vi "Trajectory Builder.vi"() -> ()   [LabVIEW 2025] (continued)
        n148 = call "Versioned Write.vi"("Path Stuff"=w308, "Filename"="Filename", "Bordeaux paths in"=w327) -> ()  [unwired: 9 in]
        n149 = Bundle("Trajectory Data"=w329, "Updated Waypoints"=w330, w328, "sorted array out"=w316) -> (w339:T27)  [unwired: 1 in]
      }
      event "Open Command": Value Change {
        # "Open Panel button was pressed. Open the subVI for the selected command"
        n150 = event-data() -> ()  [unwired: 1 in, 1 out]
        n151 = Unbundle(w372) -> ("Updated Waypoints"=w371:cluster{"x":dbl, "y":dbl, "th":dbl}[])  [unwired: 3 out]
        n152 = Unbundle(w361) -> ("Filtered Command Info Out"=w360:T2)  [unwired: 2 out]
        n153 = call "Open Command Panel.vi"("Cached Commands"=w360, "Commands"=w370, "Tag"="Command Sequence") -> ("Found"=w367:bool)  [unwired: 8 in]
        n154 = Select(t="Command Sequence", s=w367, f="") -> (s? t:f=w364:string)
        n155 = Bundle(cluster=w368, "Filename"=w364) -> (w369:T18)  [unwired: 2 in]
      }
      event "Directory": Value Change {
        # "Negate timeout to immed update list of files"
        # "Directory button was pressed. Put up a file dialog to let the user choose a new directory for loading and saving paths.\nUpdate the titlebar."
        n156 = event-data() -> ()  [unwired: 1 in, 1 out]
        n157 = Unbundle(w387) -> ("Updated Waypoints"=w386:cluster{"x":dbl, "y":dbl, "th":dbl}[])  [unwired: 3 out]
        n158 = call "File Dialog"("start path"=w382, "prompt"="Path Folder", "button label"="Select") -> ("selected path"=w381:path, "error out"=w383:errorcluster)  [unwired: 9 in, 2 out]
        n159 = Select(t=w382, s=w383, f=w381) -> (s? t:f=w375:path)
        n160 = call "Change Paths Directory.vi"("VI Refnum"=w374, "config path"=w376, "Bordeaux paths directory"=w375) -> ()  [unwired: 8 in, 1 out]
      }
      event "Delete": Value Change {
        n161 = event-data() -> ()  [unwired: 1 in, 6 out]
        n162 = Unbundle(w397) -> ("Updated Waypoints"=w396:cluster{"x":dbl, "y":dbl, "th":dbl}[])  [unwired: 3 out]
        n163 = local read "Open"() -> (w392:i32[])
        n164 = property on="Open" class="MCListbox (strict)"() -> ("ItemNames"=w394:string[][])  [unwired: 2 in, 2 out]
        n165 = Array Size(array=w392) -> (size(s)=w391:i32)
        n166 = Index Array(array=w392) -> (element=w393:i32)  [unwired: 1 in]
        n167 = Array Subset(array=w394, index (row)=w393, length (row)=w391) -> (w390:string[][])  [unwired: 2 in]
        n168 = for {
          tunnel: w390 -> [w410] mode=indexing
          tunnel: w395 -> [w411]
          n169 = Index Array(array=w410, index=0) -> (element=w404:string)
          n170 = String To Path(string=w404) -> (path=w405:path)
          n171 = Build Path(base path=w411, name or relative path=w405) -> (appended path=w408:path)
          n172 = Delete(path (use dialog)=w408, confirm (F)=FALSE) -> (error out=w406:errorcluster)  [unwired: 3 in, 2 out]
          n173 = call <vilib>:"Clear Errors.vi"("error in (no error)"=w406) -> ()  [unwired: 5 in, 2 out]
        }
      }
      event "Open": Shortcut Menu Selection (User) {
        n174 = event-data() -> ("ItemTag"=w420:string)  [unwired: 1 in, 7 out]
        n175 = case shown="\"False\", Default" w420 {
          tunnel: w419 -> [_ _ w437 _]
          tunnel: w418 -> [w427 w430 w434 w450]
          tunnel: [w426 w429 w433 w449] -> w417
          tunnel: w415 -> [w425 w428 w432 _]
          tunnel: [w425 w428 w432 w449] -> w414
          frame "False", Default {
            n176 = Unbundle(w427) -> ("Updated Waypoints"=w426:cluster{"x":dbl, "y":dbl, "th":dbl}[])  [unwired: 3 out]
          }
          frame "New Path" {
            n177 = Unbundle(w430) -> ("Updated Waypoints"=w429:cluster{"x":dbl, "y":dbl, "th":dbl}[])  [unwired: 3 out]
            n178 = local write "Conditions"(T10 {"vInitial (fps)"=0.0, "vFinal (fps)"=0.0} ("Conditions")) -> ()
          }
          frame "Delete Path(s)" {
            n179 = local read "Open"() -> (w435:i32[])
            n180 = Unbundle(w434) -> ("Updated Waypoints"=w433:cluster{"x":dbl, "y":dbl, "th":dbl}[])  [unwired: 3 out]
            n181 = property on="Open" class="MCListbox (strict)"() -> ("ItemNames"=w436:string[][])  [unwired: 2 in, 2 out]
            n182 = Array Size(array=w435) -> (size(s)=w439:i32)
            n183 = Index Array(array=w435) -> (element=w440:i32)  [unwired: 1 in]
            n184 = Array Subset(array=w436, index (row)=w440, length (row)=w439) -> (w438:string[][])  [unwired: 2 in]
            n185 = for {
              tunnel: w438 -> [w447] mode=indexing
              tunnel: w437 -> [w448]
              n186 = Index Array(array=w447, index=0) -> (element=w441:string)
              n187 = String To Path(string=w441) -> (path=w442:path)
              n188 = Build Path(base path=w448, name or relative path=w442) -> (appended path=w445:path)
              n189 = Delete(path (use dialog)=w445, confirm (F)=FALSE) -> (error out=w443:errorcluster)  [unwired: 3 in, 2 out]
              n190 = call <vilib>:"Clear Errors.vi"("error in (no error)"=w443) -> ()  [unwired: 5 in, 2 out]
            }
          }
          frame "Append to Path" {
            n191 = local read "Limits"() -> (w459:T9)
            n192 = Unbundle(w450) -> ("Updated Waypoints"=w452:cluster{"x":dbl, "y":dbl, "th":dbl}[])  [unwired: 3 out]
            n193 = local read "Conditions"() -> (w460:T10)
            n194 = Unbundle(w459) -> ("Velocity (fps)"=w454:dbl, "Accel (fps^2)"=w453:dbl)  [unwired: 2 out]
            n195 = Delete From Array(array=w452) -> (deleted portion=w457:cluster{"x":dbl, "y":dbl, "th":dbl})  [unwired: 2 in, 1 out]
            n196 = Divide(x=w454, y=w453) -> (x/y=w458:dbl)
            n197 = Build Array(w457) -> (w456:cluster{"x":dbl, "y":dbl, "th":dbl}[])
            n198 = Unbundle(w460) -> ("vFinal (fps)"=w455:dbl)  [unwired: 1 out]
            n199 = call "Add First Point.vi"("Accel (f/s^2)"=w453, "Time (s)"=w458, "Initial Points"=w456) -> ("Points"=w449:cluster{"x":dbl, "y":dbl, "th":dbl}[])  [unwired: 8 in]
            n200 = Bundle("vFinal (fps)"=w455, 0.0) -> (w461:cluster{"vFinal (fps)":dbl, dbl})  [unwired: 1 in]
            n201 = local write "Conditions"(w461) -> ()
          }
        }
      }
      event "Open": Double Click {
        # "When a path file is double clicked, load it and update the controls/indicators on the panel"
        n202 = event-data() -> ("Row"=w466:i32)  [unwired: 1 in, 8 out]
        n203 = property on="Open" class="MCListbox (strict)"() -> ("ItemNames"=w491:string[][])  [unwired: 2 in, 2 out]
        n204 = Index Array(array=w491, index (row)=w466, index (col)=0) -> (element=w467:string)
        n205 = Build Path(base path=w472, name or relative path=w467) -> (appended path=w490:path)
        n206 = local write "Filename"(w467) -> ()
        n207 = call "Versioned Load.vi"("path"=w490) -> ("Trajectory Meta"=w471:cluster{"Drive Type":T11, "Path Type":T7}, "Current Limit"=w465:dbl, "Points out"=w473:cluster{"x":dbl, "y":dbl, "th":dbl}[], "Fields"=w478:T28, "Commands out"=w484:cluster{"Time (s)":dbl, T3, bool}[], "Zero V"=w479:bool, "Ball Pickup"=w464:bool, "Reversals"=w483:T25, "Trajectory Data"=w489:T12, "Zero Translational Velocity"=w463:bool, "Correct at Beginning \nof Path"=w462:bool)  [unwired: 15 in, 1 out]
        n208 = Unbundle(w483) -> ("Robot Backwards"=w482:bool, "Reverse Path"=w481:bool)
        n209 = Unbundle(w478) -> ("Sample Period (s)"=w477:dbl, w476:T29, "Conditions"=w475:T10, "Overrides"=w474:T8)  [unwired: 1 out]
        n210 = Unbundle(w471) -> ("Drive Type"=w470:T11, "Path Type"=w469:T7)
        n211 = local write "Correct at Beginning \nof Path"(w462) -> ()
        n212 = local write "Zero Translational\n Velocity"(w463) -> ()
        n213 = local write "Current Limit"(w465) -> ()
        n214 = local write "Robot Backwards"(w482) -> ()
        n215 = local write "Zero Velocity"(w479) -> ()
        n216 = local write "Reverse Path"(w481) -> ()
        n217 = local write "Pickup Balls"(w464) -> ()
        n218 = local write "Limits"(w476) -> ()
        n219 = local write "Drive Type"(w470) -> ()
        n220 = local write "Path Type"(w469) -> ()
        n221 = local write "Sample Period (s)"(w477) -> ()
        n222 = local write "Overrides"(w474) -> ()
        n223 = local write "Conditions"(w475) -> ()
        n224 = Bundle("Trajectory Data"=w489, "Points out"=w473, "Fields"=w478, "Commands out"=w484) -> (w480:T30)  [unwired: 1 in]
      }
      event "Picture": Mouse Down {
        # "Object being clicked"
        # "Process a mouse down on the picture control. Only left clicks do anything.\nDetermine if any object was clicked on and mark it as the drag object for \nmouse move messages."
        n225 = event-data() -> ("Coords"=w506:T31, "Button"=w508:u16, "Mods"=w507:cluster{"Double Click":bool, "Menu Key":bool}, "PlatMods"=w503:T32)  [unwired: 1 in]
        n226 = Unbundle(w496) -> ("Drag Object"=w495:cluster{"Index":i32, "x":dbl, "y":dbl})  [unwired: 2 out]
        n227 = Unbundle(w500) -> ("Updated Waypoints"=w499:cluster{"x":dbl, "y":dbl, "th":dbl}[])  [unwired: 3 out]
        n228 = case shown="1" w508 {
          tunnel: w507 -> [_ _ w520]
          tunnel: w506 -> [_ _ w525]
          tunnel: w499 -> [w512 w516 w526]
          tunnel: [w512 w516 w530] -> w505
          tunnel: w504 -> [_ _ w527]
          tunnel: w495 -> [w510 w513 w521]
          tunnel: [w509 w515 w522] -> w497
          tunnel: w503 -> [_ _ w518]
          frame 0, Default {
            # "middle mouse?"
            n229 = Bundle(cluster=w510, "Index"=-1) -> (w509:cluster{"Index":i32, "x":dbl, "y":dbl})  [unwired: 2 in]
          }
          frame 2 {
            # "Right Button"
            n230 = Bundle(cluster=w513, "Index"=-1) -> (w515:cluster{"Index":i32, "x":dbl, "y":dbl})  [unwired: 2 in]
          }
          frame 1 {
            # "Left Button"
            n231 = Unbundle By Name(w520) -> ("Double Click"=w519:bool)
            n232 = property on="Picture" class="Pict"() -> ("Position"=w529:T16, "Draw Area Size"=w528:T33)  [unwired: 2 in, 2 out]
            n233 = Unbundle By Name(w518) -> ("Shift"=w517:bool)
            n234 = call "Point Test Shapes.vi"("Coords"=w525, "Points"=w526, "Picture in"=w527) -> ("Pt Test Results"=w524:enum16{"Miss", "Rect Hit", "Arrow Hit"}, "Results"=w523:T17)  [unwired: 7 in]
            n235 = case shown="\"Rect Hit\"" w524 {
              tunnel: w519 -> [_ _ w577]
              tunnel: w526 -> [w534 w562 w571]
              tunnel: w523 -> [_ w560 w578]
              tunnel: [w537 w563 w572] -> w530
              tunnel: w525 -> [w538 _ _]
              tunnel: w529 -> [w536 _ _]
              tunnel: w528 -> [w535 _ _]
              tunnel: [w532 w555 w574] -> w522
              tunnel: w521 -> [w531 _ w575]
              tunnel: w517 -> [w533 _ w567]
              frame "Miss", Default {
                n236 = case shown="True" w533 {
                  tunnel: w538 -> [w550 _]
                  tunnel: [w547 w554] -> w537
                  tunnel: w536 -> [w546 _]
                  tunnel: w535 -> [w545 _]
                  tunnel: w534 -> [w541 w554]
                  tunnel: [w540 w553] -> w532
                  tunnel: w531 -> [_ w551]
                  frame False {
                    n237 = call "Map to Feet.vi"("Draw Area Size"=w545, "Position"=w546, "Coords (px)"=w550) -> ("Point (ft)"=w544:cluster{dbl, dbl})  [unwired: 8 in]
                    n238 = Array Size(array=w541) -> (size(s)=w539:i32)
                    n239 = Unbundle(w544) -> (w543:dbl, w542:dbl)
                    n240 = Bundle(w543, w542, nan) -> (w548:cluster{dbl, dbl, dbl})  [unwired: 1 in]
                    n241 = Bundle(w539, w543, w542) -> (w540:cluster{i32, dbl, dbl})  [unwired: 1 in]
                    n242 = Build Array (concatenate)(w541, w548) -> (w547:cluster{"x":dbl, "y":dbl, "th":dbl}[])
                  }
                  frame True {
                    n243 = Bundle(cluster=w551, "Index"=-1) -> (w553:cluster{"Index":i32, "x":dbl, "y":dbl})  [unwired: 2 in]
                  }
                }
              }
              frame "Arrow Hit" {
                # "start tracking rotation"
                n244 = Unbundle(w560) -> ("Index"=w559:i32)  [unwired: 1 out]
                n245 = Index Array(array=w562, index=w559) -> (element=w561:cluster{"x":dbl, "y":dbl, "th":dbl})
                n246 = Unbundle(w561) -> ("x"=w558:dbl, "y"=w557:dbl, "th"=w565:dbl)
                n247 = Bundle(cluster=w561, "th"=w565) -> (w564:cluster{"x":dbl, "y":dbl, "th":dbl})  [unwired: 2 in]
                n248 = Bundle(-2, "x"=w558, "y"=w557) -> (w555:cluster{i32, "x":dbl, "y":dbl})  [unwired: 1 in]
                n249 = Replace Array Subset(array=w562, new element=w564) -> (w563:cluster{"x":dbl, "y":dbl, "th":dbl}[])  [unwired: 1 in]
              }
              frame "Rect Hit" {
                n250 = Unbundle(w578) -> ("Index"=w576:i32)  [unwired: 1 out]
                n251 = Array Size(array=w571) -> (size(s)=w570:i32)
                n252 = Greater?(x=w570, y=2) -> (0:w568:bool)
                n253 = And(x=w567, y=w568) -> (x .and. y?=w566:bool)
                n254 = case shown="True" w566 {
                  tunnel: w577 -> [w582 _]
                  tunnel: w576 -> [w581 w585]
                  tunnel: [w580 -1 ("length")] -> w573
                  tunnel: w571 -> [w579 w588]
                  tunnel: [w579 w587] -> w572
                  frame False {
                    n255 = case shown="False" w582 {
                      tunnel: w581 -> [w583 _]
                      tunnel: [w583 -1] -> w580
                      frame False {
                      }
                      frame True {
                        # "TODO Toggle last pt"
                      }
                    }
                  }
                  frame True {
                    n256 = case shown="0" w585 {
                      tunnel: w588 -> [w589 w593]
                      tunnel: w585 -> [_ w592]
                      tunnel: [w589 w590] -> w587
                      frame 0 {
                      }
                      frame Default {
                        n257 = Delete From Array(array=w593, length=1, index=w592) -> (array with subset deleted=w590:cluster{"x":dbl, "y":dbl, "th":dbl}[])  [unwired: 1 out]
                      }
                    }
                  }
                }
                n258 = Bundle(cluster=w575, "Index"=w573) -> (w574:cluster{"Index":i32, "x":dbl, "y":dbl})  [unwired: 2 in]
              }
            }
          }
        }
        n259 = Bundle(cluster=w496, "Drag Object"=w497) -> (w498:T18)  [unwired: 2 in]
      }
      event "Picture": Mouse Move; "Picture": Mouse Up {
        # "If an object was clicked on and is being moved, update position.\nIf nothing is being dragged, you may be hovering over an object and\nwant to draw it differently."
        n260 = event-data() -> ("Type"=w619:T21, "Coords"=w621:T31)  [unwired: 1 in]
        n261 = local read "Robot Size (in)"() -> (w601:cluster{"width":dbl, "height":dbl})
        n262 = Index Array(array=w595) -> (element=w596:cluster{"width":dbl, "height":dbl})  [unwired: 1 in]
        n263 = Unbundle By Name(w601) -> ("width"=w599:dbl)
        n264 = Unbundle By Name(w596) -> ("width"=w594:dbl)  [unwired: 1 out]
        n265 = Divide(x=w599, y=24.0) -> (x/y=w598:dbl)
        n266 = Subtract(x=w594, y=w598) -> (x-y=w597:dbl)
        n267 = Unbundle(w615) -> ("Updated Waypoints"=w614:cluster{"x":dbl, "y":dbl, "th":dbl}[])  [unwired: 3 out]
        n268 = Unbundle(w607) -> ("Drag Object"=w610:cluster{"Index":i32, "x":dbl, "y":dbl})  [unwired: 2 out]
        n269 = Unbundle(w610) -> ("Index"=w618:i32)  [unwired: 2 out]
        n270 = case shown="Default" w618 {
          selector: w618 -> [w632 _]
          tunnel: w621 -> [w641 w649]
          tunnel: [w639 w648] -> w612
          tunnel: [w636 w647] -> w620
          tunnel: w614 -> [w637 w647]
          tunnel: [w633 w646] -> w613
          tunnel: w610 -> [w624 w646]
          tunnel: w619 -> [w634 _]
          tunnel: "Snap to foot" -> [w629 _]
          tunnel: "Snap robot to baseline" -> [w630 _]
          tunnel: "Angle Limiter" -> [w631 _]
          tunnel: w606 -> [w623 w645]
          tunnel: w605 -> [_ w644]
          tunnel: w597 -> [w622 _]
          frame Default {
            # "Mouse up changes indes to break tracking,\notherwise update coords"
            n271 = property on="Picture" class="Pict"() -> ("Position"=w642:T16, "Draw Area Size"=w643:T33)  [unwired: 2 in, 2 out]
            n272 = Bundle("Snap robot to baseline"=w630, "Snap to foot"=w629, "Angle Limiter"=w631) -> (w628:T34)  [unwired: 1 in]
            n273 = Equal?(x=lveventtype."Mouse Up" ("Type"), y=w634) -> (x = y?=w627:bool)
            n274 = call "Map to Feet.vi"("Draw Area Size"=w643, "Position"=w642, "Coords (px)"=w641) -> ("Point (ft)"=w640:cluster{dbl, dbl})  [unwired: 8 in]
            n275 = call "Handle Pos and Rot.vi"("Starting Line Y"=w622, "Mouse Up"=w627, "Picture in"=w623, "Option"=w628, "Coord (ft)"=w640, "Index"=w632, "Points in"=w637) -> ("Points out"=w636:cluster{"x":dbl, "y":dbl, "th":dbl}[])  [unwired: 4 in]
            n276 = Bundle(cluster=w624, "Index"=-1) -> (w625:cluster{"Index":i32, "x":dbl, "y":dbl})  [unwired: 2 in]
            n277 = Bundle(w632, "Pt Test Results"=enum16{"Miss", "Rect Hit", "Arrow Hit"}."Rect Hit") -> (w639:T35)  [unwired: 1 in]
            n278 = Select(t=w625, s=w627, f=w624) -> (s? t:f=w633:cluster{"Index":i32, "x":dbl, "y":dbl})
          }
          frame -1 {
            n279 = call "Point Test Shapes.vi"("Array"=w644, "Coords"=w649, "Points"=w647, "Picture in"=w645) -> ("Results"=w648:T17)  [unwired: 6 in, 1 out]
          }
        }
        n280 = Bundle(cluster=w607, "Drag Object"=w613, "Hover Object"=w612) -> (w611:T18)  [unwired: 1 in]
      }
      event "Origin Reflection", "Sample Period (s)", "Horizontal Reflection", "Conditions", "Vertical Reflection": Value Change {
        # "Don't updates pts to fit rules"
        # "Changes to any of these controls will update the picture and other indicators to be consistent."
        n281 = event-data() -> ("CtlRef"=w657:refnum<vi>)  [unwired: 1 in]
        n282 = control-ref of="Vertical Reflection"() -> (w665:refnum<vi>)
        n283 = control-ref of="Origin Reflection"() -> (w658:refnum<vi>)
        n284 = control-ref of="Horizontal Reflection"() -> (w678:refnum<vi>)
        n285 = Index Array(array=w661) -> (element=w660:cluster{"width":dbl, "height":dbl})  [unwired: 1 in]
        n286 = Unbundle By Name(w660) -> ("width"=w659:dbl, "height"=w655:dbl)
        n287 = Equal?(x=w657, y=w658) -> (x = y?=w656:bool)
        n288 = Equal?(x=w678, y=w657) -> (x = y?=w663:bool)
        n289 = Equal?(x=w657, y=w665) -> (x = y?=w653:bool)
        n290 = Unbundle(w674) -> ("Updated Waypoints"=w654:cluster{"x":dbl, "y":dbl, "th":dbl}[])  [unwired: 3 out]
        n291 = case shown="True" w656 {
          tunnel: w654 -> [w679 w682]
          tunnel: [w679 w680] -> w651
          frame False {
          }
          frame True {
            n292 = Index Array(array=w682) -> (element=w681:cluster{"x":dbl, "y":dbl, "th":dbl})  [unwired: 1 in]
            n293 = for {
              tunnel: w682 -> [w700] mode=indexing
              tunnel: w681 -> [w699]
              tunnel: [w683] -> w680 mode=indexing
              n294 = Unbundle(w699) -> ("x"=w697:dbl, "y"=w695:dbl)  [unwired: 1 out]
              n295 = Unbundle(w700) -> ("x"=w693:dbl, "y"=w691:dbl, "th"=w690:dbl)
              n296 = Multiply(x=2.0, y=w697) -> (x*y=w694:dbl)
              n297 = Subtract(x=w694, y=w693) -> (x-y=w686:dbl)
              n298 = Add(x=w690, y=180.0) -> (x+y=w688:dbl)
              n299 = Multiply(x=2.0, y=w695) -> (x*y=w692:dbl)
              n300 = Quotient & Remainder(x=w688, y=360.0) -> (x-y*floor(x/y)=w684:dbl)  [unwired: 1 out]
              n301 = Subtract(x=w692, y=w691) -> (x-y=w685:dbl)
              n302 = Bundle(w686, w685, w684) -> (w683:cluster{dbl, dbl, dbl})  [unwired: 1 in]
            }
          }
        }
        n303 = case shown="True" w663 {
          tunnel: w654 -> [w716 w719]
          tunnel: [w716 w718] -> w664
          tunnel: w659 -> [_ w717]
          frame False {
          }
          frame True {
            n304 = for {
              tunnel: w719 -> [w729] mode=indexing
              tunnel: [w726] -> w718 mode=indexing
              tunnel: w717 -> [w723]
              n305 = Unbundle(w729) -> ("x"=w728:dbl, "y"=w727:dbl, "th"=w721:dbl)
              n306 = Negate(x=w728) -> (-x=w725:dbl)
              n307 = Subtract(x=180.0, y=w721) -> (x-y=w720:dbl)
              n308 = Add(x=w723, y=w725) -> (x+y=w724:dbl)
              n309 = Bundle(w724, "y"=w727, w720) -> (w726:cluster{dbl, "y":dbl, dbl})  [unwired: 1 in]
            }
          }
        }
        n310 = case shown="True" w653 {
          tunnel: w654 -> [w701 w704]
          tunnel: [w701 w703] -> w652
          tunnel: w655 -> [_ w702]
          frame False {
          }
          frame True {
            n311 = for {
              tunnel: w704 -> [w714] mode=indexing
              tunnel: [w715] -> w703 mode=indexing
              tunnel: w702 -> [w705]
              n312 = Unbundle By Name(w714) -> ("y"=w713:dbl, "x"=w712:dbl, "th"=w709:dbl)
              n313 = Negate(x=w713) -> (-x=w707:dbl)
              n314 = Negate(x=w709) -> (-x=w708:dbl)
              n315 = Add(x=w705, y=w707) -> (x+y=w706:dbl)
              n316 = Swap Values(12:w706, 14:w712) -> (1:w711:dbl, 3:w710:dbl)  [unwired: 1 in]
              n317 = Bundle(w711, w710, w708) -> (w715:cluster{dbl, dbl, dbl})  [unwired: 1 in]
            }
          }
        }
        n318 = Select(t=w652, s=w653, f=w651) -> (s? t:f=w650:cluster{"x":dbl, "y":dbl, "th":dbl}[])
        n319 = Select(t=w664, s=w663, f=w650) -> (s? t:f=w662:cluster{"x":dbl, "y":dbl, "th":dbl}[])
        n320 = local read "Path Type"() -> (w669:T7)
        n321 = case shown="\"Clothoid\", Default" w669 {
          tunnel: "Unjank" -> [_ w733]
          tunnel: w674 -> [_ w732]
          tunnel: "Turn Acceleration" -> [_ w731]
          tunnel: "Turn Deceleration" -> [_ w730]
          frame "Bezier" {
          }
          frame "Clothoid", Default {
            n322 = case shown="True" w733 {
              tunnel: w732 -> [_ w734]
              tunnel: w731 -> [_ w737]
              tunnel: w730 -> [_ w736]
              frame False {
              }
              frame True {
                n323 = call "Turn Smother.vi"("Ignore Deceleration"=w736, "Ignore Acceleration"=w737, "Internal Path Stuff"=w734) -> ("Overrides"=w735:T8)  [unwired: 1 in]
                n324 = local write "Overrides"(w735) -> ()
              }
            }
          }
        }
      }
      event Key Down?; event type 5.0.x8000000b {
        # "If hovering over an object, nudge using arrow keys"
        n325 = event-data() -> ("VKey"=w759:T36)  [unwired: 1 in]
        n326 = Index Array(array=w739) -> (element=w740:cluster{"width":dbl, "height":dbl})  [unwired: 1 in]
        n327 = local read "Robot Size (in)"() -> (w742:cluster{"width":dbl, "height":dbl})
        n328 = Unbundle By Name(w740) -> ("width"=w738:dbl)  [unwired: 1 out]
        n329 = Unbundle By Name(w742) -> ("width"=w744:dbl)
        n330 = Divide(x=w744, y=24.0) -> (x/y=w743:dbl)
        n331 = local read "Snap robot to baseline"() -> (w766:bool)
        n332 = Unbundle(w753) -> ("Updated Waypoints"=w752:cluster{"x":dbl, "y":dbl, "th":dbl}[])  [unwired: 3 out]
        n333 = Subtract(x=w738, y=w743) -> (x-y=w741:dbl)
        n334 = local read "Angle Limiter"() -> (w764:enum16{"90", "45", "15", "1"})
        n335 = local read "Snap to foot"() -> (w765:bool)
        n336 = Unbundle(w750) -> ("Hover Object"=w751:T17)  [unwired: 2 out]
        n337 = case shown="\"Up\"" w759 {
          tunnel: [cluster{dbl, dbl} {0.0, 0.0} ("Coord (ft)") cluster{dbl, dbl} {0.0, 0.1} ("Coord (ft)") cluster{dbl, dbl} {0.0, -0.1} ("Coord (ft)") cluster{dbl, dbl} {-0.1, 0.0} ("Coord (ft)") cluster{dbl, dbl} {0.1, 0.0} ("Coord (ft)")] -> w761
          tunnel: [_ w780 w782 w784 w786] -> w757
          tunnel: TRUE ("Delta") -> [_ w780 w782 w784 w786]
          frame Default {
          }
          frame "Up" {
          }
          frame "Down" {
          }
          frame "Left" {
          }
          frame "Right" {
          }
        }
        n338 = Unbundle(w751) -> ("Index"=w749:i32, "Pt Test Results"=w758:enum16{"Miss", "Rect Hit", "Arrow Hit"})
        n339 = Bundle("Snap robot to baseline"=w766, "Snap to foot"=w765, "Angle Limiter"=w764) -> (w763:T34)  [unwired: 1 in]
        n340 = case shown="\"Rect Hit\", Default" w758 {
          tunnel: [w769 w778] -> w767
          tunnel: w754 -> [_ w777]
          tunnel: w763 -> [_ w776]
          tunnel: w752 -> [w769 w775]
          tunnel: TRUE ("Delta") -> [_ w774]
          tunnel: w761 -> [_ w773]
          tunnel: w757 -> [_ w772]
          tunnel: [_ w772] -> w756
          tunnel: w749 -> [_ w771]
          tunnel: w741 -> [_ w770]
          frame "Miss" {
          }
          frame "Rect Hit", Default {
            n341 = call "Handle Pos and Rot.vi"("Starting Line Y"=w770, "Delta"=w774, "Picture in"=w777, "Option"=w776, "Coord (ft)"=w773, "Index"=w771, "Points in"=w775) -> ("Points out"=w778:cluster{"x":dbl, "y":dbl, "th":dbl}[])  [unwired: 4 in]
          }
        }
        n342 = event-data("Discard?"=w756) -> ()  [unwired: 1 in, 1 out]
      }
      event User Event {
        # "Fire events to animate the timeline\nuntil we reach the end"
        n343 = event-data() -> ("Data"=w802:i32)  [unwired: 1 in]
        n344 = Unbundle(w795) -> ("Updated Waypoints"=w794:cluster{"x":dbl, "y":dbl, "th":dbl}[])  [unwired: 3 out]
        n345 = Tick Count (ms)() -> (millisecond timer value=w805:u32)
        n346 = Subtract(x=w805, y=w802) -> (x-y=w804:u32)
        n347 = Multiply(x=w804, y=0.001) -> (x*y=w801:dbl)
        n348 = local read "Duration (s)"() -> (w788:dbl)
        n349 = Quotient & Remainder(x=w801, y=0.02) -> (floor(x/y)=w799:dbl)  [unwired: 1 out]
        n350 = Wait (ms)(milliseconds to wait=u32 50) -> ()  [unwired: 1 out]
        n351 = Multiply(x=0.02, y=w799) -> (x*y=w798:dbl)
        n352 = Less Or Equal?(x=w798, y=w788) -> (x <= y?=w807:bool)
        n353 = case shown="True" w807 {
          tunnel: w789 -> [_ w812]
          tunnel: w802 -> [_ w810]
          tunnel: w798 -> [_ w811]
          tunnel: w788 -> [w809 _]
          frame False {
            n354 = local write "Time (s)"(w809) -> ()
          }
          frame True {
            n355 = Generate User Event(user event=w812, event data cluster=w810) -> ()  [unwired: 2 in, 2 out]
            n356 = local write "Time (s)"(w811) -> ()
          }
        }
      }
      event "New Page Selector": Value Change {
        # "If looking at the commands, look at projects for one with a RIO target"
        n357 = event-data() -> ("NewVal"=w818:T1)  [unwired: 1 in]
        n358 = Unbundle(w821) -> ("Updated Waypoints"=w820:cluster{"x":dbl, "y":dbl, "th":dbl}[])  [unwired: 3 out]
        n359 = case shown="\"Command Sequencer\"" w818 {
          tunnel: [w824 w825] -> w814
          tunnel: w817 -> [w824 _]
          frame "Trajectory Settings", Default {
          }
          frame "Command Sequencer" {
            n360 = call "Find RT Projects.vi"() -> ("Paths"=w826:path[], "Targets"=w827:refnum<vi>[], "Project Names"=w828:string[])  [unwired: 9 in]
            n361 = property on="Projects" class="Ring (strict)"("Strings []"=w828) -> ()  [unwired: 2 in, 2 out]
            n362 = Bundle("Targets"=w827, "Paths"=w826) -> (w825:cluster{"Targets":refnum<vi>[], "Paths":path[]})  [unwired: 1 in]
          }
        }
        n363 = local write "Tab Control"("New Page Selector") -> ()
      }
      event "Refresh": Value Change {
        # "Refresh button was pressed. Reload the command info from the project.\nLater, maybe store this in a file because it takes awhile to recompute."
        n364 = event-data() -> ()  [unwired: 1 in, 1 out]
        n365 = Unbundle(w837) -> ("Updated Waypoints"=w836:cluster{"x":dbl, "y":dbl, "th":dbl}[])  [unwired: 3 out]
        n366 = flat-sequence {
          tunnel: [w840] -> w830
          tunnel: w832 -> [w847]
          tunnel: [w851] -> w831
          tunnel: w830 -> [w841]
          tunnel: [w841] -> w829
          tunnel: [w857] -> w834
          tunnel: w831 -> [w857]
          tunnel: w829 -> [w856]
          frame #0 {
            n367 = call <vilib>:"Set Busy.vi"() -> ("error out"=w840:errorcluster)  [unwired: 10 in, 1 out]
          }
          frame #1 {
            n368 = Unbundle(w847) -> ("Targets"=w846:refnum<vi>[], "Paths"=w845:path[])
            n369 = Index Array(array=w846, index="Projects") -> (element=w855:refnum<vi>)
            n370 = Index Array(array=w845, index="Projects") -> (element=w843:path)
            n371 = Strip Path(path=w843) -> (stripped path=w842:path)  [unwired: 1 out]
            n372 = global read "Global Settings.vi" "Icon Scale Factor"() -> (w848:dbl)
            n373 = call "Find Command Names.vi"("project root path"=w842, "TargetItem in"=w855) -> ("Paths"=w854:path[], "Command Info"=w853:T37)  [unwired: 8 in]
            n374 = call "Format Commands to Tree.vi"("Paths"=w854, "Command Info"=w853) -> ("2D Picture"=w852:picture, "Filtered Command Info Out"=w850:T2)  [unwired: 8 in]
            n375 = call "Resize Icons.vi"("Scale Factor"=w848, "Filtered Command Info Out"=w850) -> ("Filtered Command Info Out"=w849:T2)  [unwired: 9 in]
            n376 = Bundle("Filtered Command Info Out"=w849, "2D Picture"=w852, "stripped path"=w842) -> (w851:T38)  [unwired: 1 in]
            n377 = local write "Command Palette"(w852) -> ()
            n378 = local write "Cache"(w851) -> ()
          }
          frame #2 {
            n379 = call <vilib>:"Unset Busy.vi"("error in (no error)"=w856) -> ()  [unwired: 10 in, 1 out]
          }
        }
        n380 = call-poly <vilib>:"Set Cursor.vi"() -> ()  [unwired: 10 in, 2 out]
      }
      event "WayPoints": Value Change {
        # "If the waypoints control is hand-edited, pass the new data along to update the picture and other indicators\nand make it consistent"
        n381 = event-data() -> ("NewVal"=w858:cluster{"x":dbl, "y":dbl, "th":dbl}[])  [unwired: 1 in]
      }
      event event #0x53 {
        # "This is an alternative to the Inhale button. Notice that it doesn't actually modify anything at the\nmoment."
        n382 = event-data() -> ("VIName"=w868:string)  [unwired: 1 in]
        n383 = Unbundle(w878) -> ("Updated Waypoints"=w877:cluster{"x":dbl, "y":dbl, "th":dbl}[])  [unwired: 3 out]
        n384 = Unbundle(w876) -> ("Filename"=w867:string)  [unwired: 2 out]
        n385 = Search and Replace String(input string=w867, search string=w868, replace string=w868) -> (number of replacements=w873:i32)  [unwired: 5 in, 3 out]
        n386 = call "Find Command with Tag.vi"("Command Tag"=w867, "Commands"=w866) -> ("Index"=w874:i32, "Found Command"=w875:cluster{"Time (s)":dbl, T3, bool}, "Found"=w871:bool)  [unwired: 7 in]
        n387 = Not Equal To 0?(x=w873) -> (x != 0?=w872:bool)
        n388 = And(x=w871, y=w872) -> (x .and. y?=w870:bool)
        n389 = disable-structure shown="Disabled" {
          disable-tunnel: w875 -> [w886 _]
          disable-tunnel: w874 -> [w885 _]
          disable-tunnel: w870 -> [w884 _]
          disable-tunnel: [w883 _] -> w869
          disable-tunnel: w866 -> [w882 _]
          frame Disabled {
            n390 = case shown="True" w884 {
              tunnel: w886 -> [_ w893]
              tunnel: w885 -> [_ w900]
              tunnel: w882 -> [w887 w902]
              tunnel: [w887 w901] -> _
              tunnel: [_ FALSE] -> w883
              frame False {
              }
              frame True {
                n391 = Unbundle(w893) -> (w895:T3)  [unwired: 2 out]
                n392 = Unbundle(w895) -> ("Path"=w899:path)  [unwired: 6 out]
                n393 = Open VI Reference(vi path=w899) -> (vi reference=w897:refnum<vi>)  [unwired: 5 in, 1 out]
                n394 = property class="VI"(reference=w897) -> (reference out=w890:refnum<vi>, "Panel"=w898:refnum<vi>)  [unwired: 1 in, 1 out]
                n395 = property class="Pnl"(reference=w898) -> ("Controls[]"=w896:refnum<vi>[])  [unwired: 1 in, 2 out]
                n396 = for {
                  tunnel: w896 -> [w907] mode=indexing
                  tunnel: [w904] -> w894 mode=indexing
                  shift-right: [w903] -> w889
                  shift-left: w890 -> [w903]
                  n397 = property class="Ctl"(reference=w907) -> ("Label.Text"=w906:string, "Value"=w905:variant)  [unwired: 1 in, 2 out]
                  n398 = Bundle("Label.Text"=w906, "Value"=w905) -> (w904:cluster{"Label.Text":string, "Value":variant})  [unwired: 1 in]
                }
                n399 = Bundle(cluster=w895, "All Control Values Variant"=w894) -> (w892:T3)  [unwired: 6 in]
                n400 = Bundle(cluster=w893, w892) -> (w891:cluster{"Time (s)":dbl, T3, bool})  [unwired: 2 in]
                n401 = Replace Array Subset(array=w902, new element=w891, index=w900) -> (w901:cluster{"Time (s)":dbl, T3, bool}[])
                n402 = Close Reference(reference=w889) -> ()  [unwired: 1 in, 1 out]
              }
            }
          }
          frame Enabled {
          }
        }
      }
      event "Inhale": Value Change {
        # "Inhale button was pressed. Get the value of the controls/parameters and make them the\nvalues that will be used for the command."
        n403 = event-data() -> ()  [unwired: 1 in, 1 out]
        n404 = Unbundle(w919) -> ("Updated Waypoints"=w918:cluster{"x":dbl, "y":dbl, "th":dbl}[])  [unwired: 3 out]
        n405 = Unbundle(w917) -> ("Filename"=w916:string)  [unwired: 2 out]
        n406 = Unbundle(w910) -> ("Filtered Command Info Out"=w909:T2)  [unwired: 2 out]
        n407 = call "Find Command with Tag.vi"("Command Tag"=w916, "Commands"=w908) -> ("Index"=w913:i32, "Found Command"=w914:cluster{"Time (s)":dbl, T3, bool}, "Found"=w915:bool)  [unwired: 7 in]
        n408 = case shown="True" w915 {
          tunnel: w914 -> [_ w940]
          tunnel: w913 -> [_ w946]
          tunnel: w908 -> [w923 w948]
          tunnel: [w923 w947] -> w912
          tunnel: [_ TRUE] -> w911
          tunnel: w909 -> [_ w925]
          frame False {
          }
          frame True {
            n409 = Unbundle(w940) -> (w942:T3)  [unwired: 2 out]
            n410 = Unbundle(w942) -> ("Name"=w926:string, "Path"=w945:path)  [unwired: 5 out]
            n411 = Open VI Reference(vi path=w945) -> (vi reference=w927:refnum<vi>, error out=w931:errorcluster)  [unwired: 5 in]
            n412 = Unbundle(w931) -> ("code"=w930:i32)  [unwired: 2 out]
            n413 = Not Equal?(x=w930, y=0) -> (x != y?=w928:bool)
            n414 = case shown="False" w928 {
              tunnel: w927 -> [w949 w953]
              tunnel: w926 -> [_ w952]
              tunnel: w925 -> [_ w951]
              tunnel: [w949 w950] -> w924
              frame False {
              }
              frame True {
                n415 = call "Replace Command with Cached Command.vi"("Cached Commands"=w951, "Name"=w952, "VI in"=w953) -> ("VI out"=w950:refnum<vi>)  [unwired: 8 in]
              }
            }
            n416 = property class="VI"(reference=w924) -> (reference out=w937:refnum<vi>, "Panel"=w944:refnum<vi>)  [unwired: 1 in, 1 out]
            n417 = property class="Pnl"(reference=w944) -> (reference out=w935:refnum<vi>, "Controls[]"=w943:refnum<vi>[])  [unwired: 1 in, 1 out]
            n418 = for {
              tunnel: w943 -> [w959] mode=indexing
              tunnel: [w956] -> w941 mode=indexing
              shift-right: [w955] -> w934
              shift-left: w937 -> [w955]
              shift-right: [w954] -> _
              shift-left: w935 -> [w954]
              n419 = property class="Ctl"(reference=w959) -> ("Label.Text"=w958:string, "Value"=w957:variant)  [unwired: 1 in, 2 out]
              n420 = Bundle("Label.Text"=w958, "Value"=w957) -> (w956:cluster{"Label.Text":string, "Value":variant})  [unwired: 1 in]
            }
            n421 = Bundle(cluster=w942, "All Control Values Variant"=w941) -> (w939:T3)  [unwired: 6 in]
            n422 = Bundle(cluster=w940, w939) -> (w938:cluster{"Time (s)":dbl, T3, bool})  [unwired: 2 in]
            n423 = Replace Array Subset(array=w948, new element=w938, index=w946) -> (w947:cluster{"Time (s)":dbl, T3, bool}[])
            n424 = property class="VI"(reference=w934, "FP.State"=T22."Closed" ("Front Panel Window:State")) -> (reference out=w933:refnum<vi>)  [unwired: 1 in, 1 out]
            n425 = Close Reference(reference=w933) -> ()  [unwired: 1 in, 1 out]
          }
        }
      }
      event "fps": Cursor Move {
        # "The red cursor on the velocity graph was moved to a new location. Update the time slider to be in sync"
        n426 = event-data() -> ("CursIdx"=w962:i32, "CursLoc"=w968:cluster{"X":dbl, "Y":dbl})  [unwired: 1 in]
        n427 = Unbundle(w969) -> ("Updated Waypoints"=w967:cluster{"x":dbl, "y":dbl, "th":dbl}[])  [unwired: 3 out]
        n428 = Array Size(array=w965) -> (size(s)=w964:i32)
        n429 = Greater?(x=w964, y=w962) -> (0:w963:bool)
        n430 = case shown="False" w963 {
          tunnel: w968 -> [w976 w981]
          tunnel: w965 -> [w974 w979]
          tunnel: [w974 w978] -> w966
          tunnel: w962 -> [_ w977]
          frame False {
            n431 = Unbundle(w976) -> ("X"=w975:dbl)  [unwired: 1 out]
            n432 = local write "Time (s)"(w975) -> ()
          }
          frame True {
            n433 = Unbundle(w981) -> ("X"=w980:dbl)  [unwired: 1 out]
            n434 = in-place {
              in-place-border: w980 -> [w984]
              n435 = in-place-array #2(w979, w977) -> (w983:cluster{"Time (s)":dbl, T3, bool})
              n436 = Bundle(cluster=w983, "Time (s)"=w984) -> (w982:cluster{"Time (s)":dbl, T3, bool})  [unwired: 2 in]
              n437 = in-place-array #2(w982) -> (w978:cluster{"Time (s)":dbl, T3, bool}[])  [unwired: 1 out]
            }
          }
        }
      }
      event "Command Sequence": Mouse Down {
        # "second column, tag starting with // indicates an enable click"
        # "Handle a click on a row of the tree within the Command Sequencer tab.\nThis only handles the enable/disable click"
        n438 = event-data() -> ("CtlRef"=w999:refnum<vi>, "Coords"=w1000:T31, "PlatMods.Shift"=w985:bool)  [unwired: 1 in]
        n439 = Unbundle(w1002) -> ("Updated Waypoints"=w1001:cluster{"x":dbl, "y":dbl, "th":dbl}[])  [unwired: 3 out]
        n440 = invoke class="Tree (strict)" method="Point To Row Column"(reference=w999, "Point"=w1000) -> ("Tag"=w990:string, "Col"=w994:i32)  [unwired: 6 in, 6 out]
        n441 = String Subset(string=w990, length (rest)=2 ("length (rest)")) -> (substring=w998:string)  [unwired: 1 in]
        n442 = Equal?(x=2 ("length (rest)"), y=w994) -> (x = y?=w993:bool)
        n443 = Equal?(x="//", y=w998) -> (x = y?=w992:bool)
        n444 = And(x=w992, y=w993) -> (x .and. y?=w991:bool)
        n445 = case shown="True" w991 {
          tunnel: w989 -> [w1007 w1010]
          tunnel: w990 -> [_ w1014]
          tunnel: [w1007 w1009] -> w987
          tunnel: [_ TRUE] -> w988
          tunnel: w985 -> [_ w1008]
          frame False {
          }
          frame True {
            # "click on enable of a command"
            n446 = call "Find Command with Tag.vi"("Command Tag"=w1014, "Commands"=w1010) -> ("Index"=w1011:i32, "Found Command"=w1012:cluster{"Time (s)":dbl, T3, bool}, "Found"=w1013:bool)  [unwired: 7 in]
            n447 = case shown="False" w1008 {
              tunnel: w1013 -> [w1020 _]
              tunnel: w1012 -> [w1019 _]
              tunnel: w1011 -> [w1018 w1029]
              tunnel: w1010 -> [w1017 w1032]
              tunnel: [w1016 w1031] -> w1009
              frame False {
                # "Toggle"
                n448 = case shown="True" w1020 {
                  tunnel: w1019 -> [_ w1023]
                  tunnel: w1018 -> [_ w1026]
                  tunnel: w1017 -> [w1021 w1027]
                  tunnel: [w1021 w1024] -> w1016
                  frame False {
                  }
                  frame True {
                    n449 = Unbundle(w1023) -> (w1022:bool)  [unwired: 2 out]
                    n450 = Not(x=w1022) -> (.not. x?=w1028:bool)
                    n451 = Bundle(cluster=w1023, w1028) -> (w1025:cluster{"Time (s)":dbl, T3, bool})  [unwired: 2 in]
                    n452 = Replace Array Subset(array=w1027, new element=w1025, index=w1026) -> (w1024:cluster{"Time (s)":dbl, T3, bool}[])
                  }
                }
              }
              frame True {
                # "Delete"
                n453 = Delete From Array(array=w1032, length=1, index=w1029) -> (array with subset deleted=w1031:cluster{"Time (s)":dbl, T3, bool}[])  [unwired: 1 out]
              }
            }
          }
        }
      }
      event "Command Sequence": Double Click {
        # "This handles a double-click of a command in the first column. This opens the panel \nand updates the parameters to the values in the command."
        n454 = event-data() -> ("CtlRef"=w1048:refnum<vi>, "Coords"=w1049:T31)  [unwired: 1 in]
        n455 = Unbundle(w1051) -> ("Updated Waypoints"=w1050:cluster{"x":dbl, "y":dbl, "th":dbl}[])  [unwired: 3 out]
        n456 = invoke class="Tree (strict)" method="Point To Row Column"(reference=w1048, "Point"=w1049) -> ("Tag"=w1038:string, "Col"=w1043:i32)  [unwired: 6 in, 6 out]
        n457 = String Subset(string=w1038, length (rest)=2 ("length (rest)")) -> (substring=w1047:string)  [unwired: 1 in]
        n458 = Equal?(x=0 ("length (rest)"), y=w1043) -> (x = y?=w1042:bool)
        n459 = Equal?(x="//", y=w1047) -> (x = y?=w1041:bool)
        n460 = And(x=w1041, y=w1042) -> (x .and. y?=w1040:bool)
        n461 = Unbundle(w1034) -> ("Filtered Command Info Out"=w1033:T2)  [unwired: 2 out]
        n462 = case shown="True" w1040 {
          tunnel: w1039 -> [_ w1060]
          tunnel: w1038 -> [_ w1058]
          tunnel: [_ w1057] -> w1035
          tunnel: w1033 -> [_ w1055]
          frame False {
          }
          frame True {
            n463 = call "Open Command Panel.vi"("Cached Commands"=w1055, "Commands"=w1060, "Tag"=w1058) -> ("Found"=w1059:bool)  [unwired: 8 in]
            n464 = Select(t=w1058, s=w1059, f="") -> (s? t:f=w1057:string)
          }
        }
        n465 = Bundle(cluster=w1036, "Filename"=w1035) -> (w1037:T18)  [unwired: 2 in]
      }
      event "Command Sequence": Edit Cell? {
        # "This allows you to enter time  directly using the tree cell"
        n466 = event-data() -> ("String"=w1069:string, "Tag"=w1068:string, "Col"=w1071:i32)  [unwired: 1 in]
        n467 = Unbundle(w1078) -> ("Updated Waypoints"=w1077:cluster{"x":dbl, "y":dbl, "th":dbl}[])  [unwired: 3 out]
        n468 = Equal?(x=1 ("length (rest)"), y=w1071) -> (x = y?=w1072:bool)
        n469 = String Subset(string=w1068, length (rest)=2 ("length (rest)")) -> (substring=w1076:string)  [unwired: 1 in]
        n470 = Equal?(x="//", y=w1076) -> (x = y?=w1073:bool)
        n471 = And(x=w1073, y=w1072) -> (x .and. y?=w1070:bool)
        n472 = case shown="True" w1070 {
          tunnel: [TRUE _] -> w1064
          tunnel: w1069 -> [_ w1092]
          tunnel: w1066 -> [w1083 w1089]
          tunnel: w1068 -> [_ w1088]
          tunnel: [w1083 w1090] -> w1062
          frame False {
          }
          frame True {
            n473 = call "Find Command with Tag.vi"("Command Tag"=w1088, "Commands"=w1089) -> ("Index"=w1086:i32, "Found Command"=w1085:cluster{"Time (s)":dbl, T3, bool}, "Found"=w1087:bool)  [unwired: 7 in]
            n474 = Scan From String(input string=w1092) -> (output 1=w1091:dbl)  [unwired: 4 in, 3 out]
            n475 = case shown="True" w1087 {
              tunnel: w1089 -> [w1093 w1096]
              tunnel: [w1093 w1097] -> w1090
              tunnel: w1091 -> [_ w1098]
              tunnel: w1086 -> [_ w1094]
              tunnel: w1085 -> [_ w1099]
              frame False {
              }
              frame True {
                n476 = Bundle(cluster=w1099, "Time (s)"=w1098) -> (w1095:cluster{"Time (s)":dbl, T3, bool})  [unwired: 2 in]
                n477 = Replace Array Subset(array=w1096, new element=w1095, index=w1094) -> (w1097:cluster{"Time (s)":dbl, T3, bool}[])
              }
            }
          }
        }
        n478 = Sort 1D Array(array=w1062) -> (sorted array=w1061:cluster{"Time (s)":dbl, T3, bool}[])
        n479 = Not(x=w1064) -> (.not. x?=w1065:bool)
        n480 = event-data("Discard?"=w1064) -> ()  [unwired: 1 in, 1 out]
      }
      event "Command Palette": Mouse Move {
        # "Draw the hilite for the row that the mouse is over"
        n481 = event-data() -> ("Coords"=w1107:T31)  [unwired: 1 in]
        n482 = Unbundle(w1110) -> ("Updated Waypoints"=w1109:cluster{"x":dbl, "y":dbl, "th":dbl}[])  [unwired: 3 out]
        n483 = control-ref of="Command Palette"() -> (w1103:refnum<vi>)
        n484 = call "Picture Coord to Row.vi"("Row Height"=w1102, "Coords"=w1107, "Picture in"=w1103) -> ("Row Index"=w1104:i32, "Clicked in canvas"=w1106:bool)  [unwired: 7 in]
        n485 = Unbundle(w1100) -> ("Filtered Command Info Out"=w1105:T2, "2D Picture"=w1108:picture)  [unwired: 1 out]
        n486 = case shown="True" w1106 {
          tunnel: w1108 -> [_ w1118]
          tunnel: w1105 -> [_ _]
          tunnel: w1102 -> [_ w1116]
          tunnel: w1104 -> [_ w1115]
          frame False {
          }
          frame True {
            n487 = Multiply(x=w1115, y=w1116) -> (x*y=w1121:i32)
            n488 = Add(x=w1121, y=w1116) -> (x+y=w1122:i32)
            n489 = Bundle(0, w1121, 300, w1122) -> (w1123:cluster{i32, i32, i32, i32})  [unwired: 1 in]
            n490 = call <vilib>:"Draw Rectangle.vi"("rect"=w1123, "fill?(F)"=TRUE, "color(black)"=u32 10539263) -> ("new picture"=w1125:picture)  [unwired: 6 in]
            n491 = Concatenate Strings(w1125, w1118) -> (→"Command Palette":picture)
          }
        }
      }
      event "Command Palette": Mouse Down {
        # "When a double click occurs in the command palette,\nadd the command to the command list at time T."
        n492 = event-data() -> ("Coords"=w1137:T31, "Mods"=w1139:cluster{"Double Click":bool, "Menu Key":bool})  [unwired: 1 in, 1 out]
        n493 = control-ref of="Command Palette"() -> (w1138:refnum<vi>)
        n494 = Unbundle(w1141) -> ("Updated Waypoints"=w1140:cluster{"x":dbl, "y":dbl, "th":dbl}[])  [unwired: 3 out]
        n495 = call "Picture Coord to Row.vi"("Row Height"=w1136, "Coords"=w1137, "Picture in"=w1138) -> ("Row Index"=w1132:i32, "Clicked in canvas"=w1135:bool)  [unwired: 7 in]
        n496 = Unbundle(w1139) -> ("Double Click"=w1134:bool)  [unwired: 1 out]
        n497 = Unbundle(w1128) -> ("Filtered Command Info Out"=w1131:T2)  [unwired: 2 out]
        n498 = Compound Arithmetic op=AND(w1135, w1134) -> (w1133:bool)
        n499 = case shown="True" w1133 {
          tunnel: w1132 -> [_ w1153]
          tunnel: w1131 -> [_ w1154]
          tunnel: w1130 -> [w1146 w1148]
          tunnel: [w1146 w1149] -> w1127
          frame False {
          }
          frame True {
            n500 = local read "Time (s)"() -> (w1150:dbl)
            n501 = Index Array(array=w1154, index=w1153) -> (element=w1152:T3)
            n502 = Bundle("Time (s)"=w1150, w1152, TRUE) -> (w1147:cluster{"Time (s)":dbl, T3, bool})  [unwired: 1 in]
            n503 = call "Insert Into Sorted Array.vim"("element"=w1147, "sorted array in"=w1148) -> ("sorted array out"=w1149:cluster{"Time (s)":dbl, T3, bool}[])  [unwired: 9 in]
          }
        }
      }
    }
    n504 = feedback-in #1(w98) -> ()
    n505 = Unbundle(w73) -> (w72:T14)  [unwired: 3 out]
    n506 = Unbundle(w72) -> ("Limits"=w74:T9)  [unwired: 4 out]
    n507 = Unbundle(w74) -> ("Velocity (fps)"=w71:dbl)  [unwired: 3 out]